vi "SaccadeAnalyser - Main.vi"(8 "error in (no error)":errorcluster, 11 "Data IN":T3={"Impulse Positions"=[{"Start"=5471, "End"=5813, "Impulse Plane"=enum."Yaw", "Impulse Direction +ve?"=FALSE, "Time offset"=0, "Amplitude offset"=0.0}, {"Start"=6974, "End"=7325, "Impulse Plane"=enum."Yaw", "Impulse Direction +ve?"=TRUE, "Time offset"=0, "Amplitude offset"=0.0}, {"Start"=7641, "End"=7980, "Impulse Plane"=enum."Yaw", "Impulse Direction +ve?"=FALSE, "Time offset"=0, "Amplitude offset"=0.0}, {"Start"=9060, "End"=9400, "Impulse Plane"=enum."Yaw", "Impulse Direction +ve?"=FALSE, "Time offset"=0, "Amplitude offset"=0.0}, {"Start"=9938, "End"=10282, "Impulse Plane"=enum."Yaw", "Impulse Direction +ve?"=FALSE, "Time offset"=0, "Amplitude offset"=0.0}, {"Start"=10800, "End"=11142, "Impulse Plane"=enum."Yaw", "Impulse Direction +ve?"=FALSE, "Time offset"=0, "Amplitude offset"=0.0}, {"Start"=11602, "End"=11942, "Impulse Plane"=enum."Yaw", "Impulse Direction +ve?"=TRUE, "Time offset"=0, "Amplitude offset"=0.0}, {"Start"=12449, "End"=12790, "Impulse Plane"=enum."Yaw", "Impulse Direction +ve?"=TRUE, "Time offset"=0, "Amplitude offset"=0.0}, {"Start"=13310, "End"=13653, "Impulse Plane"=enum."Yaw", "Impulse Direction +ve?"=TRUE, "Time offset"=0, "Amplitude offset"=0.0}, {"Start"=14191, "End"=14535, "Impulse Plane"=enum."Yaw", "Impulse Direction +ve?"=TRUE, "Time offset"=0, "Amplitude offset"=0.0}, {"Start"=15040, "End"=15380, "Impulse Plane"=enum."Yaw", "Impulse Direction +ve?"=FALSE, "Time offset"=0, "Amplitude offset"=0.0}, {"Start"=16780, "End"=17124, "Impulse Plane"=enum."Yaw", "Impulse Direction +ve?"=TRUE, "Time offset"=0, "Amplitude offset"=0.0}, {"Start"=17572, "End"=17913, "Impulse Plane"=enum."Yaw", "Impulse Direction +ve?"=FALSE, "Time offset"=0, "Amplitude offset"=0.0}, {"Start"=18369, "End"=18713, "Impulse Plane"=enum."Yaw", "Impulse Direction +ve?"=FALSE, "Time offset"=0, "Amplitude offset"=0.0}, {"Start"=19174, "End"=19519, "Impulse Plane"=enum."Yaw", "Impulse Direction +ve?"=FALSE, "Time offset"=0, "Amplitude offset"=0.0}, {"Start"=19928, "End"=20270, "Impulse Plane"=enum."Yaw", "Impulse Direction +ve?"=TRUE, "Time offset"=0, "Amplitude offset"=0.0}, {"Start"=20762, "End"=21121, "Impulse Plane"=enum."Yaw", "Impulse Direction +ve?"=FALSE, "Time offset"=0, "Amplitude offset"=0.0}, {"Start"=21554, "End"=21888, "Impulse Plane"=enum."Yaw", "Impulse Direction +ve?"=FALSE, "Time offset"=0, "Amplitude offset"=0.0}, {"Start"=22293, "End"=22639, "Impulse Plane"=enum."Yaw", "Impulse Direction +ve?"=TRUE, "Time offset"=0, "Amplitude offset"=0.0}, {"Start"=23109, "End"=23464, "Impulse Plane"=enum."Yaw", "Impulse Direction +ve?"=TRUE, "Time offset"=0, "Amplitude offset"=0.0}, {"Start"=23868, "End"=24215, "Impulse Plane"=enum."Yaw", "Impulse Direction +ve?"=TRUE, "Time offset"=0, "Amplitude offset"=0.0}, {"Start"=24643, "End"=24992, "Impulse Plane"=enum."Yaw", "Impulse Direction +ve?"=FALSE, "Time offset"=0, "Amplitude offset"=0.0}, {"Start"=25685, "End"=26023, "Impulse Plane"=enum."Yaw", "Impulse Direction +ve?"=FALSE, "Time offset"=0, "Amplitude offset"=0.0}, {"Start"=26431, "End"=26768, "Impulse Plane"=enum."Yaw", "Impulse Direction +ve?"=FALSE, "Time offset"=0, "Amplitude offset"=0.0}, {"Start"=27251, "End"=27595, "Impulse Plane"=enum."Yaw", "Impulse Direction +ve?"=FALSE, "Time offset"=0, "Amplitude offset"=0.0}, {"Start"=28832, "End"=29180, "Impulse Plane"=enum."Yaw", "Impulse Direction +ve?"=TRUE, "Time offset"=0, "Amplitude offset"=0.0}, {"Start"=31028, "End"=31383, "Impulse Plane"=enum."LARP", "Impulse Direction +ve?"=FALSE, "Time offset"=0, "Amplitude offset"=0.0}, {"Start"=32603, "End"=32936, "Impulse Plane"=enum."LARP", "Impulse Direction +ve?"=TRUE, "Time offset"=0, "Amplitude offset"=0.0}, {"Start"=33445, "End"=33779, "Impulse Plane"=enum."LARP", "Impulse Direction +ve?"=TRUE, "Time offset"=0, "Amplitude offset"=0.0}, {"Start"=34276, "End"=34629, "Impulse Plane"=enum."LARP", "Impulse Direction +ve?"=FALSE, "Time offset"=0, "Amplitude offset"=0.0}, {"Start"=35114, "End"=35460, "Impulse Plane"=enum."LARP", "Impulse Direction +ve?"=FALSE, "Time offset"=0, "Amplitude offset"=0.0}, {"Start"=35981, "End"=36324, "Impulse Plane"=enum."LARP", "Impulse Direction +ve?"=TRUE, "Time offset"=0, "Amplitude offset"=0.0}, {"Start"=36920, "End"=37249, "Impulse Plane"=enum."LARP", "Impulse Direction +ve?"=TRUE, "Time offset"=0, "Amplitude offset"=0.0}, {"Start"=37988, "End"=38322, "Impulse Plane"=enum."LARP", "Impulse Direction +ve?"=TRUE, "Time offset"=0, "Amplitude offset"=0.0}, {"Start"=38964, "End"=39324, "Impulse Plane"=enum."LARP", "Impulse Direction +ve?"=FALSE, "Time offset"=0, "Amplitude offset"=0.0}, {"Start"=39948, "End"=40284, "Impulse Plane"=enum."LARP", "Impulse Direction +ve?"=TRUE, "Time offset"=0, "Amplitude offset"=0.0}, {"Start"=40958, "End"=41293, "Impulse Plane"=enum."LARP", "Impulse Direction +ve?"=TRUE, "Time offset"=0, "Amplitude offset"=0.0}, {"Start"=41899, "End"=42229, "Impulse Plane"=enum."LARP", "Impulse Direction +ve?"=TRUE, "Time offset"=0, "Amplitude offset"=0.0}, {"Start"=42801, "End"=43154, "Impulse Plane"=enum."LARP", "Impulse Direction +ve?"=FALSE, "Time offset"=0, "Amplitude offset"=0.0}, {"Start"=43641, "End"=43980, "Impulse Plane"=enum."LARP", "Impulse Direction +ve?"=TRUE, "Time offset"=0, "Amplitude offset"=0.0}, {"Start"=44466, "End"=44821, "Impulse Plane"=enum."LARP", "Impulse Direction +ve?"=FALSE, "Time offset"=0, "Amplitude offset"=0.0}, {"Start"=45388, "End"=45722, "Impulse Plane"=enum."LARP", "Impulse Direction +ve?"=TRUE, "Time offset"=0, "Amplitude offset"=0.0}, {"Start"=46149, "End"=46510, "Impulse Plane"=enum."LARP", "Impulse Direction +ve?"=FALSE, "Time offset"=0, "Amplitude offset"=0.0}, {"Start"=47874, "End"=48206, "Impulse Plane"=enum."LARP", "Impulse Direction +ve?"=TRUE, "Time offset"=0, "Amplitude offset"=0.0}, {"Start"=50143, "End"=50479, "Impulse Plane"=enum."RALP", "Impulse Direction +ve?"=TRUE, "Time offset"=0, "Amplitude offset"=0.0}, {"Start"=50976, "End"=51310, "Impulse Plane"=enum."RALP", "Impulse Direction +ve?"=FALSE, "Time offset"=0, "Amplitude offset"=0.0}, {"Start"=51892, "End"=52226, "Impulse Plane"=enum."RALP", "Impulse Direction +ve?"=FALSE, "Time offset"=0, "Amplitude offset"=0.0}, {"Start"=52839, "End"=53171, "Impulse Plane"=enum."RALP", "Impulse Direction +ve?"=FALSE, "Time offset"=0, "Amplitude offset"=0.0}, {"Start"=53676, "End"=54012, "Impulse Plane"=enum."RALP", "Impulse Direction +ve?"=TRUE, "Time offset"=0, "Amplitude offset"=0.0}, {"Start"=54530, "End"=54877, "Impulse Plane"=enum."RALP", "Impulse Direction +ve?"=FALSE, "Time offset"=0, "Amplitude offset"=0.0}, {"Start"=55371, "End"=55711, "Impulse Plane"=enum."RALP", "Impulse Direction +ve?"=TRUE, "Time offset"=0, "Amplitude offset"=0.0}, {"Start"=56153, "End"=56482, "Impulse Plane"=enum."RALP", "Impulse Direction +ve?"=FALSE, "Time offset"=0, "Amplitude offset"=0.0}, {"Start"=57053, "End"=57390, "Impulse Plane"=enum."RALP", "Impulse Direction +ve?"=FALSE, "Time offset"=0, "Amplitude offset"=0.0}, {"Start"=57954, "End"=58292, "Impulse Plane"=enum."RALP", "Impulse Direction +ve?"=FALSE, "Time offset"=0, "Amplitude offset"=0.0}, {"Start"=58794, "End"=59130, "Impulse Plane"=enum."RALP", "Impulse Direction +ve?"=TRUE, "Time offset"=0, "Amplitude offset"=0.0}, {"Start"=59587, "End"=59931, "Impulse Plane"=enum."RALP", "Impulse Direction +ve?"=TRUE, "Time offset"=0, "Amplitude offset"=0.0}, {"Start"=60399, "End"=60744, "Impulse Plane"=enum."RALP", "Impulse Direction +ve?"=FALSE, "Time offset"=0, "Amplitude offset"=0.0}, {"Start"=61218, "End"=61559, "Impulse Plane"=enum."RALP", "Impulse Direction +ve?"=FALSE, "Time offset"=0, "Amplitude offset"=0.0}, {"Start"=62100, "End"=62442, "Impulse Plane"=enum."RALP", "Impulse Direction +ve?"=FALSE, "Time offset"=0, "Amplitude offset"=0.0}, {"Start"=62989, "End"=63322, "Impulse Plane"=enum."RALP", "Impulse Direction +ve?"=FALSE, "Time offset"=0, "Amplitude offset"=0.0}, {"Start"=63787, "End"=64136, "Impulse Plane"=enum."RALP", "Impulse Direction +ve?"=TRUE, "Time offset"=0, "Amplitude offset"=0.0}, {"Start"=64603, "End"=64953, "Impulse Plane"=enum."RALP", "Impulse Direction +ve?"=FALSE, "Time offset"=0, "Amplitude offset"=0.0}, {"Start"=65462, "End"=65795, "Impulse Plane"=enum."RALP", "Impulse Direction +ve?"=FALSE, "Time offset"=0, "Amplitude offset"=0.0}, {"Start"=66308, "End"=66645, "Impulse Plane"=enum."RALP", "Impulse Direction +ve?"=FALSE, "Time offset"=0, "Amplitude offset"=0.0}, {"Start"=67052, "End"=67402, "Impulse Plane"=enum."RALP", "Impulse Direction +ve?"=TRUE, "Time offset"=0, "Amplitude offset"=0.0}], "No. Imp"=15, "Parameter Time Series"=[{"time offset"=0.0, "Offset"=0.0, "Gain"=1.0, "inverse"=FALSE, "filter data"=FALSE, "dots"=FALSE, "interpolate"=FALSE, "List 1"=5, "Color Box"=6618880, "Boolean"=TRUE}, {"time offset"=0.0, "Offset"=0.0, "Gain"=1.0, "inverse"=FALSE, "filter data"=FALSE, "dots"=FALSE, "interpolate"=FALSE, "List 1"=6, "Color Box"=6618880, "Boolean"=FALSE}, {"time offset"=0.0, "Offset"=0.0, "Gain"=1.0, "inverse"=FALSE, "filter data"=FALSE, "dots"=FALSE, "interpolate"=FALSE, "List 1"=7, "Color Box"=6618880, "Boolean"=FALSE}, {"time offset"=0.0, "Offset"=0.0, "Gain"=1.0, "inverse"=FALSE, "filter data"=FALSE, "dots"=FALSE, "interpolate"=FALSE, "List 1"=13, "Color Box"=16777224, "Boolean"=TRUE}, {"time offset"=0.0, "Offset"=0.0, "Gain"=1.0, "inverse"=FALSE, "filter data"=FALSE, "dots"=FALSE, "interpolate"=FALSE, "List 1"=14, "Color Box"=16777224, "Boolean"=FALSE}, {"time offset"=0.0, "Offset"=0.0, "Gain"=1.0, "inverse"=FALSE, "filter data"=FALSE, "dots"=FALSE, "interpolate"=FALSE, "List 1"=15, "Color Box"=16777224, "Boolean"=FALSE}], "Parameter Impuls Series"=[{"Color"=6618880, "Visible"=TRUE, "Channel"=1, "Invert"=FALSE, "Desaccade"=FALSE, "Offset"=0.0, "Gain"=1.0}, {"Color"=6618880, "Visible"=FALSE, "Channel"=6, "Invert"=FALSE, "Desaccade"=FALSE, "Offset"=0.0, "Gain"=1.0}, {"Color"=6618880, "Visible"=FALSE, "Channel"=7, "Invert"=FALSE, "Desaccade"=FALSE, "Offset"=0.0, "Gain"=1.0}, {"Color"=16777224, "Visible"=TRUE, "Channel"=13, "Invert"=FALSE, "Desaccade"=FALSE, "Offset"=0.0, "Gain"=1.0}, {"Color"=16777224, "Visible"=FALSE, "Channel"=14, "Invert"=FALSE, "Desaccade"=FALSE, "Offset"=0.0, "Gain"=1.0}, {"Color"=16777224, "Visible"=FALSE, "Channel"=15, "Invert"=FALSE, "Desaccade"=FALSE, "Offset"=0.0, "Gain"=1.0}], "Experiment Parameters"={"Freq"=0.0, "Vel"=0, "Acc"=0, "Stimulus"="Head Impulse"}, "Autosort File"=refnum, "Data File"={"Data Channels"=array34x71049[2415666 elements], "Sample Rate"=500, "Channel List"=["Hz Position-in-Head", "Hz Velocity-in-Head", "Hy Position-in-Head", "Hy Velocity-in-Head", "Hx Position-in-Head", "Hx Velocity-in-Head", "Hl Velocity-in-Head", "Hr Velocity-in-Head", "Lx Position-in-Head", "Ly Position-in-Head", "Lz Position-in-Head", "Lx Velocity-in-Head", "Ly Velocity-in-Head", "Lz Velocity-in-Head", "Ll Velocity-in-Head", "Lr Velocity-in-Head", "Rx Position-in-Head", "Ry Position-in-Head", "Rz Position-in-Head", "Rx Velocity-in-Head", "Ry Velocity-in-Head", "Rz Velocity-in-Head", "Rl Velocity-in-Head", "Rr Velocity-in-Head", "Target on/off", "aux input 1", "aux input 2", " ", "", "", "", "Target Hor", "Target Ver", ""]}, "Experiment data path"=path "C:/Users/w.figtree/Desktop/Coils Data/3", "Image data path"=path "/Macintosh HD/Users/patrick/Studium/Diploma Thesis/Data Analysis", "LVS data path"=path "/Macintosh HD/Users/patrick/Studium/Diploma Thesis/Data Analysis", "Raw copy path"=path "/Macintosh HD/Users/patrick/Studium/Diploma Thesis/Data Analysis", "filename"="passive_lvs.lvs", "desaccading parameters"={"Tolerance"=3, "Acc Range"=7000.0, "Sample Rate"=500, "Impulse Plane 2"=enum."Yaw", "Impulse dir"=FALSE}, "Experiment Parameters 2"={"Subject"="SE Trial Short Term", "Strain"="", "Rotation plane"="", "Experimenter"=" ", "Trial"=0.0, "Time"=0.0}, "Excel"={"Excel._Application"=refnum, "Use Excel"=TRUE, "Worksheet SINE"=refnum, "Row SINE"=0, "Worksheet TRANS"=refnum, "Row TRANS"=0}, "Session Config File"=refnum, "Autosort Parameter Set"=4, "EMA Version"="EMA 2016a", "desacc "={"Threshold 1 [Acc]"=7000.0, "Threshold 2 [% of TH1]"=60, "tolerance"=3, "Search WD "=0.1, " always use TH2"=FALSE, "Range"=3.0, "Max time"=120.0, "Min time"=20.0, "Velocity Threshold"=150}, "Cycle Nr for Saccades"={"POS"=0, "NEG"=0}, "calibration name"="u_calibration_1_p00001s001_calib.mat", "Excel"=refnum} {"Parameter Time Series"."time offset" format="%.3f"; "Parameter Time Series"."Gain" format="%.1f"; "Parameter Time Series"."Offset" format="%.1f"; "Parameter Time Series"."List 1" items=["Motor-Pos", "Motor-Vel", "Lx Position-in-Head", "Ly Position-in-Head", "Lz Position-in-Head", "Lx Velocity-in-Head", "Ly Velocity-in-Head", "Lz Velocity-in-Head", "Ll Velocity-in-Head", "Lr Velocity-in-Head", "Lx Accel-in-Head", "Ly Accel-in-Head", "Lz Accel-in-Head", "Rx Position-in-Head", "Ry Position-in-Head", "Rz Position-in-Head", "Rx Velocity-in-Head", "Ry Velocity-in-Head", "Rz Velocity-in-Head", "Rl Velocity-in-Head", "Rr Velocity-in-Head", "Rx Accel-in-Head", "Ry Accel-in-Head", "Rz Accel-in-Head", "Global Trigger", "", "", ""]; "Parameter Impuls Series"."Gain" format="%.1f"; "Parameter Impuls Series"."Offset" format="%.1f"}) -> (0 "error out":errorcluster, 3 "Data OUT":T3={"Impulse Positions"=[{"Start"=5471, "End"=5813, "Impulse Plane"=enum."Yaw", "Impulse Direction +ve?"=FALSE, "Time offset"=0, "Amplitude offset"=0.0}, {"Start"=6974, "End"=7325, "Impulse Plane"=enum."Yaw", "Impulse Direction +ve?"=TRUE, "Time offset"=0, "Amplitude offset"=0.0}, {"Start"=7641, "End"=7980, "Impulse Plane"=enum."Yaw", "Impulse Direction +ve?"=FALSE, "Time offset"=0, "Amplitude offset"=0.0}, {"Start"=9060, "End"=9400, "Impulse Plane"=enum."Yaw", "Impulse Direction +ve?"=FALSE, "Time offset"=0, "Amplitude offset"=0.0}, {"Start"=9938, "End"=10282, "Impulse Plane"=enum."Yaw", "Impulse Direction +ve?"=FALSE, "Time offset"=0, "Amplitude offset"=0.0}, {"Start"=10800, "End"=11142, "Impulse Plane"=enum."Yaw", "Impulse Direction +ve?"=FALSE, "Time offset"=0, "Amplitude offset"=0.0}, {"Start"=11602, "End"=11942, "Impulse Plane"=enum."Yaw", "Impulse Direction +ve?"=TRUE, "Time offset"=0, "Amplitude offset"=0.0}, {"Start"=12449, "End"=12790, "Impulse Plane"=enum."Yaw", "Impulse Direction +ve?"=TRUE, "Time offset"=0, "Amplitude offset"=0.0}, {"Start"=13310, "End"=13653, "Impulse Plane"=enum."Yaw", "Impulse Direction +ve?"=TRUE, "Time offset"=0, "Amplitude offset"=0.0}, {"Start"=14191, "End"=14535, "Impulse Plane"=enum."Yaw", "Impulse Direction +ve?"=TRUE, "Time offset"=0, "Amplitude offset"=0.0}, {"Start"=15040, "End"=15380, "Impulse Plane"=enum."Yaw", "Impulse Direction +ve?"=FALSE, "Time offset"=0, "Amplitude offset"=0.0}, {"Start"=16780, "End"=17124, "Impulse Plane"=enum."Yaw", "Impulse Direction +ve?"=TRUE, "Time offset"=0, "Amplitude offset"=0.0}, {"Start"=17572, "End"=17913, "Impulse Plane"=enum."Yaw", "Impulse Direction +ve?"=FALSE, "Time offset"=0, "Amplitude offset"=0.0}, {"Start"=18369, "End"=18713, "Impulse Plane"=enum."Yaw", "Impulse Direction +ve?"=FALSE, "Time offset"=0, "Amplitude offset"=0.0}, {"Start"=19174, "End"=19519, "Impulse Plane"=enum."Yaw", "Impulse Direction +ve?"=FALSE, "Time offset"=0, "Amplitude offset"=0.0}, {"Start"=19928, "End"=20270, "Impulse Plane"=enum."Yaw", "Impulse Direction +ve?"=TRUE, "Time offset"=0, "Amplitude offset"=0.0}, {"Start"=20762, "End"=21121, "Impulse Plane"=enum."Yaw", "Impulse Direction +ve?"=FALSE, "Time offset"=0, "Amplitude offset"=0.0}, {"Start"=21554, "End"=21888, "Impulse Plane"=enum."Yaw", "Impulse Direction +ve?"=FALSE, "Time offset"=0, "Amplitude offset"=0.0}, {"Start"=22293, "End"=22639, "Impulse Plane"=enum."Yaw", "Impulse Direction +ve?"=TRUE, "Time offset"=0, "Amplitude offset"=0.0}, {"Start"=23109, "End"=23464, "Impulse Plane"=enum."Yaw", "Impulse Direction +ve?"=TRUE, "Time offset"=0, "Amplitude offset"=0.0}, {"Start"=23868, "End"=24215, "Impulse Plane"=enum."Yaw", "Impulse Direction +ve?"=TRUE, "Time offset"=0, "Amplitude offset"=0.0}, {"Start"=24643, "End"=24992, "Impulse Plane"=enum."Yaw", "Impulse Direction +ve?"=FALSE, "Time offset"=0, "Amplitude offset"=0.0}, {"Start"=25685, "End"=26023, "Impulse Plane"=enum."Yaw", "Impulse Direction +ve?"=FALSE, "Time offset"=0, "Amplitude offset"=0.0}, {"Start"=26431, "End"=26768, "Impulse Plane"=enum."Yaw", "Impulse Direction +ve?"=FALSE, "Time offset"=0, "Amplitude offset"=0.0}, {"Start"=27251, "End"=27595, "Impulse Plane"=enum."Yaw", "Impulse Direction +ve?"=FALSE, "Time offset"=0, "Amplitude offset"=0.0}, {"Start"=28832, "End"=29180, "Impulse Plane"=enum."Yaw", "Impulse Direction +ve?"=TRUE, "Time offset"=0, "Amplitude offset"=0.0}, {"Start"=31028, "End"=31383, "Impulse Plane"=enum."LARP", "Impulse Direction +ve?"=FALSE, "Time offset"=0, "Amplitude offset"=0.0}, {"Start"=32603, "End"=32936, "Impulse Plane"=enum."LARP", "Impulse Direction +ve?"=TRUE, "Time offset"=0, "Amplitude offset"=0.0}, {"Start"=33445, "End"=33779, "Impulse Plane"=enum."LARP", "Impulse Direction +ve?"=TRUE, "Time offset"=0, "Amplitude offset"=0.0}, {"Start"=34276, "End"=34629, "Impulse Plane"=enum."LARP", "Impulse Direction +ve?"=FALSE, "Time offset"=0, "Amplitude offset"=0.0}, {"Start"=35114, "End"=35460, "Impulse Plane"=enum."LARP", "Impulse Direction +ve?"=FALSE, "Time offset"=0, "Amplitude offset"=0.0}, {"Start"=35981, "End"=36324, "Impulse Plane"=enum."LARP", "Impulse Direction +ve?"=TRUE, "Time offset"=0, "Amplitude offset"=0.0}, {"Start"=36920, "End"=37249, "Impulse Plane"=enum."LARP", "Impulse Direction +ve?"=TRUE, "Time offset"=0, "Amplitude offset"=0.0}, {"Start"=37988, "End"=38322, "Impulse Plane"=enum."LARP", "Impulse Direction +ve?"=TRUE, "Time offset"=0, "Amplitude offset"=0.0}, {"Start"=38964, "End"=39324, "Impulse Plane"=enum."LARP", "Impulse Direction +ve?"=FALSE, "Time offset"=0, "Amplitude offset"=0.0}, {"Start"=39948, "End"=40284, "Impulse Plane"=enum."LARP", "Impulse Direction +ve?"=TRUE, "Time offset"=0, "Amplitude offset"=0.0}, {"Start"=40958, "End"=41293, "Impulse Plane"=enum."LARP", "Impulse Direction +ve?"=TRUE, "Time offset"=0, "Amplitude offset"=0.0}, {"Start"=41899, "End"=42229, "Impulse Plane"=enum."LARP", "Impulse Direction +ve?"=TRUE, "Time offset"=0, "Amplitude offset"=0.0}, {"Start"=42801, "End"=43154, "Impulse Plane"=enum."LARP", "Impulse Direction +ve?"=FALSE, "Time offset"=0, "Amplitude offset"=0.0}, {"Start"=43641, "End"=43980, "Impulse Plane"=enum."LARP", "Impulse Direction +ve?"=TRUE, "Time offset"=0, "Amplitude offset"=0.0}, {"Start"=44466, "End"=44821, "Impulse Plane"=enum."LARP", "Impulse Direction +ve?"=FALSE, "Time offset"=0, "Amplitude offset"=0.0}, {"Start"=45388, "End"=45722, "Impulse Plane"=enum."LARP", "Impulse Direction +ve?"=TRUE, "Time offset"=0, "Amplitude offset"=0.0}, {"Start"=46149, "End"=46510, "Impulse Plane"=enum."LARP", "Impulse Direction +ve?"=FALSE, "Time offset"=0, "Amplitude offset"=0.0}, {"Start"=47874, "End"=48206, "Impulse Plane"=enum."LARP", "Impulse Direction +ve?"=TRUE, "Time offset"=0, "Amplitude offset"=0.0}, {"Start"=50143, "End"=50479, "Impulse Plane"=enum."RALP", "Impulse Direction +ve?"=TRUE, "Time offset"=0, "Amplitude offset"=0.0}, {"Start"=50976, "End"=51310, "Impulse Plane"=enum."RALP", "Impulse Direction +ve?"=FALSE, "Time offset"=0, "Amplitude offset"=0.0}, {"Start"=51892, "End"=52226, "Impulse Plane"=enum."RALP", "Impulse Direction +ve?"=FALSE, "Time offset"=0, "Amplitude offset"=0.0}, {"Start"=52839, "End"=53171, "Impulse Plane"=enum."RALP", "Impulse Direction +ve?"=FALSE, "Time offset"=0, "Amplitude offset"=0.0}, {"Start"=53676, "End"=54012, "Impulse Plane"=enum."RALP", "Impulse Direction +ve?"=TRUE, "Time offset"=0, "Amplitude offset"=0.0}, {"Start"=54530, "End"=54877, "Impulse Plane"=enum."RALP", "Impulse Direction +ve?"=FALSE, "Time offset"=0, "Amplitude offset"=0.0}, {"Start"=55371, "End"=55711, "Impulse Plane"=enum."RALP", "Impulse Direction +ve?"=TRUE, "Time offset"=0, "Amplitude offset"=0.0}, {"Start" (continued)
0.3136463359014541, 0.8356439558190694, 1.0807730511591118, 1.008152579414918, 0.6403622918618552, 0.05726854459087516, -0.6226124016069239, -1.2683049046170205, -1.760683781141545, -2.0210161355059197, -2.027835760987729, -1.8073040771073665, -1.421770309430135, -0.9580303700049866, -0.497301313900923, -0.09616678522946565, 0.21452094700539082, 0.4282575940550948, 0.5538563498224214, 0.6021705911165827, 0.5818891930397305, 0.48953386690155987, 0.3063405176033549, 0.015461762921761935, -0.3964258317397493, -0.9249482868494889, -1.540268926057795, -2.2073725916132383, -2.8846320076226544, -3.538587091438709, -4.158197240468231, -4.7531153797235435, -5.364891718192799, -6.052061560219654, -6.874949289764504, -7.897233446082333, -9.171337740143038, -10.72488328045902, -12.562414766990466, -14.67457205858573, -17.045384715402072, -19.654868304000217, -22.49134409148419, -25.555765096573193, -28.85378979168178, -32.39596723967773, -36.19203959960508, -40.23604923396587, -44.50374011243326, -48.95861277984851, -53.54945363728179, -58.22156929857021, -62.93553580494907, -67.66786295001663, -72.41299041244334, -77.18792215364881, -82.02000309278964, -86.92685719919085, -91.90104121434112, -96.90878594721156, -101.89052876496476, -106.75742086199175, -111.41385146978266, -115.77939241062663, -119.79675861338215, -123.4483336844591, -126.76745878295363, -129.8197559088528, -132.6790937391208, -135.42118601104028, -138.09732315600553, -140.7075535824381, -143.20185487348436, -145.48994066966543, -147.45225959610104, -148.9562412522947, -149.88438536669352, -150.15938999946377, -149.7551185366133, -148.7055372942553, -147.0966779613204, -145.05100616289218, -142.7084564262063, -140.19315566583424, -137.59376966259333, -134.95409526921003, -132.2621545061447, -129.45532916363223, -126.44396629750773, -123.14306685808681, -119.49322221297906, -115.46765411034396, -111.09174770085767, -106.43650985129578, -101.59132800894649, -96.65438967293429, -91.71259435775372, -86.8192692202177, -82.00231506366208, -77.2733493277404, -72.62220379415442, -68.04066017480889, -63.53900609944821, -59.13502207662985, -54.85489044963556, -50.73212183918571, -46.793187335728675, -43.048655658168116, -39.490455930708094, -36.09811476366343, -32.84582268161397, -29.707697290358908, -26.67259343005773, -23.747244649043203, -20.952779842519245, -18.320924933671574, -15.886823028625077, -13.678249997677776, -11.706071389153173, -9.967474467452258, -8.449484224398718, -7.131560344789376, -5.9875177127288275, -4.989475816950337, -4.114309560845022, -3.343730605782561, -2.6636316967386016, -2.0689325730927393, -1.5643120394501313, -1.1589236901372326, -0.8692686011417561, -0.7160895083609655, -0.7043677558509762, -0.8125319466466728, -0.998603306700675, -1.2005617105084991, -1.33531101092179, -1.3160973471338342, -1.0809687945741104, -0.6120433072437053, 0.06340754891936085, 0.8749545158033338, 1.715030095203367, 2.4693795282274738, 3.046705420730314, 3.389835847988852, 3.4926790594391433, 3.4082356614488627, 3.2207138351883113, 3.0222467554293777, 2.9008273141722585, 2.9113702994460136, 3.06230335915953, 3.3242152738387163, 3.643793639492993, 3.9574761526255755, 4.208999257845501, 4.365650588020905, 4.430592628941358, 4.436932345814542, 4.425205126791875, 4.436515958939433, 4.498281460714364, 4.612570709441531, 4.757416159199121, 4.896014364031479, 4.997320150747733, 5.043711721731824, 5.034732395497959, 4.991600326435557, 4.950353355989492, 4.94125922148622, 4.979748868652162, 5.070637000179872, 5.19840768558464, 5.329311550819548, 5.4288752009126116, 5.470495244660439, 5.444446435702417, 5.36392154071315, 5.252131142489729, 5.136094877020704, 5.044557456368848, 4.997552601671427, 5.005073910819104, 5.062786317537216, 5.151134255913403, 5.240869814798977, 5.298432314481547, 5.298794718900588, 5.231852910826348, 5.099324967656705, 4.916611294016909, 4.711103890319216, 4.517065884391753, 4.368683836714396, 4.2906441385731915, 4.298872435900009, 4.398287130030789, 4.580516924446378, 4.82709405477779, 5.107151899300531, 5.380976558125089, 5.61099355897168, 5.765535324266579, 5.819936676411081, 5.765346513854819, 5.612543635732611, 5.3935923287010565, 5.152775243612803, 4.9257125842021985, 4.737207059293002, 4.594090274181161, 4.477209549434265, 4.34707543556661, 4.165269468814407, 3.914439256723525, 3.5964364263191344, 3.2419194867797296, 2.9078456649380686, 2.6561395942611767, 2.531982281268591, 2.546331818055377, 2.6703318478912657, 2.834343552562386, 2.944708875670918, 2.9050522099993925, 2.6389790237890405, 2.12671302975548, 1.418889250283371, 0.6238736915728023, -0.11039366524286987, -0.6308505180382777, -0.8151700879495758, -0.597803895840542, 0.0070055367271688596, 0.895210597248802, 1.8897480939404439, 2.7911231199140616, 3.416880648116873, 3.6300682621946585, 3.3802602303567273, 2.714286339055203, 1.756240979107572, 0.6829891093729543, -0.3083806490161862, -1.0479984245147556, -1.4312586561845482, -1.4347089991094446, -1.1160682892110607, -0.5972213740033059, -0.03837846422525182, 0.4022063984773432, 0.6154284176945577, 0.5633943724000154, 0.28036849241931705, -0.13640386558643414, -0.5545213634049535, -0.8393255053487625, -0.8878051494774866, -0.6654594812819123, -0.2112426885811427, 0.38202708039910505, 0.984953026815937, 1.4606396010293796, 1.7129564248377385, 1.7104169406288268, 1.4806220937248753, 1.1146683785851472, 0.7439374706219706, 0.4966413541787542, 0.4768864327505309, 0.748557603534902, 1.3161416989650583, 2.1231292291711448, 3.078635720471638, 4.0798230333926, 5.025016058534048, 5.837743811293767, 6.481394899162784, 6.960851169589428, 7.31091542134686, 7.576504300818475, 7.80215065254667, 8.025213056512872, 8.266729486449622, 8.520017400763797, 8.754927161059008, 8.940703497230391, 9.042968842100333, 9.029365329703811, 8.889804260691243, 8.629142733263894, 8.270950168903735, 7.856884120767749, 7.437881513601069]}, {[0.0, 2.0, 4.0, 6.0, 8.0, 10.0, 12.0, 14.0, 16.0, 18.000000000000004, 20.0, 22.0, 24.0, 26.000000000000004, 28.0, 30.0, 32.0, 34.0, 36.00000000000001, 38.0, 40.0, 42.0, 44.0, 46.0, 48.0, 50.0, 52.00000000000001, 54.0, 56.0, 58.0, 60.0, 62.0, 64.0, 66.0, 68.0, 70.0, 72.00000000000001, 74.0, 76.0, 78.0, 80.0, 82.0, 84.0, 86.0, 88.0, 90.0, 92.0, 94.0, 96.0, 98.0, 100.0, 102.00000000000001, 104.00000000000001, 106.0, 108.0, 110.0, 112.0, 114.0, 116.0, 118.00000000000001, 120.0, 122.0, 124.0, 126.0, 128.0, 130.0, 132.0, 134.0, 136.0, 138.0, 140.0, 142.00000000000003, 144.00000000000003, 146.0, 148.0, 150.0, 152.0, 154.0, 156.0, 158.0, 160.0, 162.0, 164.0, 166.0, 168.0, 170.0, 172.0, 174.00000000000003, 176.0, 178.0, 180.0, 182.0, 184.0, 186.0, 188.0, 190.0, 192.0, 194.0, 196.0, 198.0, 200.0, 202.0, 204.00000000000003, 206.00000000000003, 208.00000000000003, 210.0, 212.0, 214.0, 216.0, 218.0, 220.0, 222.0, 224.0, 226.0, 228.0, 230.0, 232.0, 234.0, 236.00000000000003, 238.00000000000003, 240.0, 242.0, 244.0, 246.0, 248.0, 250.0, 252.0, 254.0, 256.0, 258.0, 260.0, 262.0, 264.0, 266.0, 268.0, 270.0, 272.0, 274.0, 276.0, 278.0, 280.0, 282.0, 284.00000000000006, 286.00000000000006, 288.00000000000006, 290.0, 292.0, 294.0, 296.0, 298.0, 300.0, 302.0, 304.0, 306.0, 308.0, 310.0, 312.0, 314.0, 316.0, 318.0, 320.0, 322.0, 324.0, 326.0, 328.0, 330.0, 332.0, 334.0, 336.0, 338.0, 340.0, 342.0, 344.0, 346.00000000000006, 348.00000000000006, 350.00000000000006, 352.0, 354.0, 356.0, 358.0, 360.0, 362.0, 364.0, 366.0, 368.0, 370.0, 372.0, 374.0, 376.0, 378.0, 380.0, 382.0, 384.0, 386.0, 388.0, 390.0, 392.0, 394.0, 396.0, 398.0, 400.0, 402.0, 404.0, 406.0, 408.00000000000006, 410.00000000000006, 412.00000000000006, 414.00000000000006, 416.00000000000006, 418.0, 420.0, 422.0, 424.0, 426.0, 428.0, 430.0, 432.0, 434.0, 436.0, 438.0, 440.0, 442.0, 444.0, 446.0, 448.0, 450.0, 452.0, 454.0, 456.0, 458.0, 460.0, 462.0, 464.0, 466.0, 468.0, 470.00000000000006, 472.00000000000006, 474.00000000000006, 476.00000000000006, 478.00000000000006, 480.0, 482.0, 484.0, 486.0, 488.0, 490.0, 492.0, 494.0, 496.0, 498.0, 500.0, 502.0, 504.0, 506.0, 508.0, 510.0, 512.0, 514.0, 516.0, 518.0, 520.0, 522.0, 524.0, 526.0, 528.0, 530.0, 532.0, 534.0, 536.0, 538.0, 540.0, 542.0, 544.0, 546.0, 548.0, 550.0, 552.0, 554.0, 556.0, 558.0, 560.0, 562.0, 564.0, 566.0000000000001, 568.0000000000001, 570.0000000000001, 572.0000000000001, 574.0000000000001, 576.0000000000001, 578.0, 580.0, 582.0, 584.0, 586.0, 588.0, 590.0, 592.0, 594.0, 596.0, 598.0, 600.0, 602.0, 604.0, 606.0, 608.0, 610.0, 612.0, 614.0, 616.0, 618.0, 620.0, 622.0, 624.0, 626.0, 628.0, 630.0, 632.0, 634.0, 636.0, 638.0, 640.0, 642.0, 644.0, 646.0, 648.0, 650.0, 652.0, 654.0, 656.0, 658.0, 660.0, 662.0, 664.0, 666.0, 668.0], [-0.7268796579571344, 0.5868756400558155, 1.849061589300014, 2.8955072949001277, 3.5938092667891013, 3.8706086644180715, 3.718786982722172, 3.1946415300213644, 2.407282185824542, 1.4912008254490559, 0.5809558618665704, -0.21002920069113173, -0.7939402634577206, -1.1045483177196864, -1.103397716304599, -0.7753241091748393, -0.14607692054291732, 0.6923105835593724, 1.586185761251155, 2.3265081945670367, 2.67383108173906, 2.4321740316685947, 1.5290994874503454, 0.09229891236648413, -1.4877826026253764, -2.5780618818949375, -2.392799053057046, -0.14430099606653446, 4.746702057922544, 12.452602523092203, 22.60344854279237, 34.25757503645384, 46.01122127385558, 56.22099063678715, 63.29901158559194, 66.03047497139923, 63.832602241310155, 56.889011749532884, 46.12475327143588, 33.03357630928615, 19.39626069465463, 6.9410766371388455, -2.9577672161239086, -9.480695270979776, -12.448846241585766, -12.266601981809778, -9.753870531818134, -5.927052630643125, -1.7807320869450203, 1.8839452348351586, 4.563112495256811, 6.068134677940779, 6.478298781913548, 6.048530744049282, 5.115658717067058, 4.017173043438252, 3.021697028150713, 2.3016823430805213, 1.9437130665771232, 1.9672245235198211, 2.3335946718142506, 2.9641392203780526, 3.7712619520762094, 4.669375262333061, 5.581483477253853, 6.455888373996665, 7.253822089154301, 7.941604054074936, 8.506693892586522, 8.956706892902282, 9.307963372595207, 9.593713633536598, 9.869348419224412, 10.202813907860328, 10.678039126437993, 11.387166036037426, 12.42126877594724, 13.870646130716276, 15.798105571020539, 18.220910732916984, 21.117305578571152, 24.417088654835098, 28.00453134371605, 31.74146476716203, 35.4901032652717, 39.14450505294441, 42.655837512261485, 46.04481145910139, 49.39680035672849, 52.85321050270352, 56.589749557125835, 60.77417843719481, 65.53657108555919, 70.94784313666247, 77.00213341122146, 83.62132912680406, 90.6700353525156, 97.97155408391009, 105.32762816097002, 112.55055670568973, 119.49565650805312, 126.05788476449914, 132.17532134282033, 137.84419076945738, 143.11960776620052, 148.09692542538977, 152.88535084897768, 157.59573420367354, 162.33083272603898, 167.17058153944774, 172.1420740537937, 177.21283829245147, 182.30190303576782, 187.2838960933783, 192.01403431557333, 196.348728676037, 200.1554853479829, 203.332999086979, 205.8275706086613, 207.632053225805, 208.76643957420453, 209.27071689631157, 209.20416799703486, 208.62702221972052, 207.59444083769398, 206.15596268947883, 204.3507693221406, 202.2096559605813, 199.7338712007981, 196.8818127108662, 193.58952780500164, 189.7802908198958, 185.3760543362304, 180.3170608615727, 174.59314296701893, 168.2737158327031, 161.50331599957605, 154.4864865707927, 147.454790900415, 140.62070327293839, 134.1437610991673, 128.10352303745614, 122.4736003260162, 117.13249166898223, 111.90734540979449, 106.605823800602, 101.06066958049949, 95.16443227474969, 88.88213798244476, 82.26676390616939, 75.44169074275362, 68.5558067116721, 61.7534561231178, 55.15977959362588, 48.865103227657016, 42.908454570336744, 37.280407713595196, 31.939978344845954, 26.831398654521458, 21.903737695002587, 17.118961249538277, 12.463035538071795, 7.946846855220585, 3.604096068173268, -0.5023819518888946, -4.3043374478698935, -7.742978121131118, -10.777559986626533, -13.405559508089022, -15.66254808943221, -17.61749754024314, -19.36822290377573, -21.01572327656443, -22.63076739081007, -24.242997513339702, -25.833402742867744, -27.326294531964603, -28.61020025411165, -29.573711400276494, -30.13803796876091, -30.277781235905028, -30.031601713344877, -29.49536781269699, -28.809625778264454, -28.131942380632903, -27.590090131045226, -27.254798825198392, -27.12763444164021, -27.148001673595793, -27.21631801583282, -27.218267782920297, -27.059605556145616, -26.703125143869258, -26.16770242269404, -25.513186572431987, -24.836172156350983, -24.23518392535658, -23.77532502644087, -23.475879842548103, -23.300381910500214, -23.175719393626295, -23.020569864711582, -22.762476619133928, -22.360396165090044, -21.822738074179547, -21.203221846632154, -20.58073431873988, -20.04404279102951, -19.666128843574402, -19.480358555205466, -19.48161044136967, -19.625224811468023, -19.834505045533266, -20.015541501462096, -20.06996998487608, -19.920030464294143, -19.520665997815073, -18.86651904906851, -18.00086145984146, -17.00379278662555, -15.972772195030286, -15.015447840136948, -14.231261588736627, -13.67584118566892, -13.353075503143431, -13.214025560294441, -13.155312001941855, -13.05261375167065, -12.78435555004259, -12.248525872326002, -11.40214259608435, -10.27752125240556, -8.95808243229831, -7.560924222034636, -6.220073578226758, -5.049147962104105, -4.114383544020147, -3.426933704912157, -2.9541793124894022, -2.63622739510173, -2.4049980356701193, -2.2097440844579372, -2.026116360955192, -1.855338787764457, -1.715271186082175, -1.620272862162726, -1.5660955215208876, -1.5242639070713606, -1.4450987028506148, -1.2668873015531386, -0.9508250963845928, -0.5044604903854086, 0.02374202749303045, 0.5453091688958391, 0.9465761504366021, 1.1219277427916374, 0.9984102752747752, 0.552827089574027, -0.1693160125783102, -1.0657071207847189, -2.0100113635743284, -2.879279135891757, -3.5775926520055847, -4.051880723729383, -4.299243904480527, -4.355769535922203, -4.282165464073977, -4.1551129042327055, -4.0451521592187305, -3.9930232689231744, -4.011151333409908, -4.089414119775753, -4.190481970143164, -4.266174365399207, -4.281759340004578, -4.229513166498258, -4.1506343303568265, -4.148308998453023, -4.365275353565227, -4.934751803823243, -5.942584823808536, -7.38191683807639, -9.080046765081676, -10.678128490411645, -11.6707704891704, -11.469856027373027, -9.5158355327974, -5.413075001297588, 0.9434399127670785, 9.27089343229068, 18.885806355145963, 28.78298155221996, 37.772096486182164, 44.65829905955033, 48.46266031046852, 48.61309811323283, 45.03993832436139, 38.180486368387854, 28.912453408573064, 18.402759339239452, 7.886075499642308, -1.5232402772824392, -8.985318767842745, -14.04591575558494, -16.647938966841256, -17.078934812254147, -15.873611988630202, -13.67825841551836, -11.126693516226487, -8.75133974901441, -6.914469835107074, -5.79130915420498, -5.392496893963983, -5.604907953876882, -6.254276829625091, -7.149358122125852, -8.11159996147794, -9.008475816853233, -9.767450438189652, -10.355876857063658, -10.767424091566273, -11.02576021977282, -11.168196469998328, -11.226776643595022, -11.222867460412607, -11.167808577043974, -11.069052677104303, -10.923331040952524, -10.720601583070183, -10.450978001577495, -10.104285703995224, -9.684066294686541, -9.201259838192332, -8.67246523913766]}, {[0.0, 2.0, 4.0, 6.0, 8.0, 10.0, 12.0, 14.0, 16.0, 18.000000000000004, 20.0, 22.0, 24.0, 26.000000000000004, 28.0, 30.0, 32.0, 34.0, 36.00000000000001, 38.0, 40.0, 42.0, 44.0, 46.0, 48.0, 50.0, 52.00000000000001, 54.0, 56.0, 58.0, 60.0, 62.0, 64.0, 66.0, 68.0, 70.0, 72.00000000000001, 74.0, 76.0, 78.0, 80.0, 82.0, 84.0, 86.0, 88.0, 90.0, 92.0, 94.0, 96.0, 98.0, 100.0, 102.00000000000001, 104.00000000000001, 106.0, 108.0, 110.0, 112.0, 114.0, 116.0, 118.00000000000001, 120.0, 122.0, 124.0, 126.0, 128.0, 130.0, 132.0, 134.0, 136.0, 138.0, 140.0, 142.00000000000003, 144.00000000000003, 146.0, 148.0, 150.0, 152.0, 154.0, 156.0, 158.0, 160.0, 162.0, 164.0, 166.0, 168.0, 170.0, 172.0, 174.00000000000003, 176.0, 178.0, 180.0, 182.0, 184.0, 186.0, 188.0, 190.0, 192.0, 194.0, 196.0, 198.0, 200.0, 202.0, 204.00000000000003, 206.00000000000003, 208.00000000000003, 210.0, 212.0, 214.0, 216.0, 218.0, 220.0, 222.0, 224.0, 226.0, 228.0, 230.0, 232.0, 234.0, 236.00000000000003, 238.00000000000003, 240.0, 242.0, 244.0, 246.0, 248.0, 250.0, 252.0, 254.0, 256.0, 258.0, 260.0, 262.0, 264.0, 266.0, 268.0, 270.0, 272.0, 274.0, 276.0, 278.0, 280.0, 282.0, 284.00000000000006, 286.00000000000006, 288.00000000000006, 290.0, 292.0, 294.0, 296.0, 298.0, 300.0, 302.0, 304.0, 306.0, 308.0, 310.0, 312.0, 314.0, 316.0, 318.0, 320.0, 322.0, 324.0, 326.0, 328.0, 330.0, 332.0, 334.0, 336.0, 338.0, 340.0, 342.0, 344.0, 346.00000000000006, 348.00000000000006, 350.00000000000006, 352.0, 354.0, 356.0, 358.0, 360.0, 362.0, 364.0, 366.0, 368.0, 370.0, 372.0, 374.0, 376.0, 378.0, 380.0, 382.0, 384.0, 386.0, 388.0, 390.0, 392.0, 394.0, 396.0, 398.0, 400.0, 402.0, 404.0, 406.0, 408.00000000000006, 410.00000000000006, 412.00000000000006, 414.00000000000006, 416.00000000000006, 418.0, 420.0, 422.0, 424.0, 426.0, 428.0, 430.0, 432.0, 434.0, 436.0, 438.0, 440.0, 442.0, 444.0, 446.0, 448.0, 450.0, 452.0, 454.0, 456.0, 458.0, 460.0, 462.0, 464.0, 466.0, 468.0, 470.00000000000006, 472.00000000000006, 474.00000000000006, 476.00000000000006, 478.00000000000006, 480.0, 482.0, 484.0, 486.0, 488.0, 490.0, 492.0, 494.0, 496.0, 498.0, 500.0, 502.0, 504.0, 506.0, 508.0, 510.0, 512.0, 514.0, 516.0, 518.0, 520.0, 522.0, 524.0, 526.0, 528.0, 530.0, 532.0, 534.0, 536.0, 538.0, 540.0, 542.0, 544.0, 546.0, 548.0, 550.0, 552.0, 554.0, 556.0, 558.0, 560.0, 562.0, 564.0, 566.0000000000001, 568.0000000000001, 570.0000000000001, 572.0000000000001, 574.0000000000001, 576.0000000000001, 578.0, 580.0, 582.0, 584.0, 586.0, 588.0, 590.0, 592.0, 594.0, 596.0, 598.0, 600.0, 602.0, 604.0, 606.0, 608.0, 610.0, 612.0, 614.0, 616.0, 618.0, 620.0, 622.0, 624.0, 626.0, 628.0, 630.0, 632.0, 634.0, 636.0, 638.0, 640.0, 642.0, 644.0, 646.0, 648.0, 650.0, 652.0, 654.0, 656.0, 658.0, 660.0, 662.0, 664.0, 666.0, 668.0], [-0.9294200725299575, -1.6617912267075283, -2.352385582131326, -2.913374193277157, -3.2655491322785366, -3.3578230132737446, -3.178791674604284, -2.760029313225317, -2.168722405873517, -1.492535179713748, -0.820663011357226, -0.22334144559465585, 0.2555260989539505, 0.5962038607675169, 0.798059760170279, 0.8619927604515283, 0.7879198562017748, 0.5758794795792319, 0.21700350768576016, -0.29167132882843205, -0.9283864297384028, -1.6401312663848522, -2.342077200658121, -2.9294637545298734, -3.299014224929506, -3.3716516365625395, -3.118164538425807, -2.5776961705106682, -1.8510978328465857, -1.0814042326723703, -0.4234053373937572, -0.007881036716877787, 0.08231743351444809, -0.1669912154922879, -0.691965340112787, -1.3677626147922335, -2.0407963594089065, -2.564960231382586, -2.83184946210115, -2.7953929254337027, -2.4839069529762465, -1.9836700207824376, -1.4180141921602996, -0.9265325515244469, -0.6281012244094502, -0.5975653434205244, -0.8561926537645501, -1.3663845221250652, -2.04220506774434, -2.7685360025527377, -3.421464474108137, -3.8944916086980603, -4.124038130630039, -4.093396470363512, -3.8367459814956124, -3.4330065869708086, -2.9822742333976677, -2.588431048939767, -2.3439850445162187, -2.3185117078293427, -2.5436851787803847, -3.0102088316778914, -3.6813166756743976, -4.499078717403875, -5.394722889320697, -6.303700990591801, -7.162984086821801, -7.915424334486153, -8.526498669574494, -8.983637441763289, -9.291319756838089, -9.476618324159103, -9.595511233304197, -9.726947586345972, -9.963458679537766, -10.403153823572271, -11.140256785056206, -12.257777520765012, -13.810652915492552, -15.815630641323594, -18.255813255170345, -21.080006248588028, -24.211021323518683, -27.56203343046876, -31.053007430265353, -34.62774040826604, -38.26448725938374, -41.980809209974595, -45.823594486609856, -49.862747452460006, 